vi "HFRR ADV v040 new software.vi"() -> ()   [LabVIEW 2025] (continued)
          frame False {
          }
          frame True {
            n1303 = Not(x=w1625) -> (.not. x?=w1624:bool)
            n1304 = local write "LIVE FEED MIN TEMP"(w1624) -> ()
            n1305 = call "CAMERA LIVE FEED FGV.vi"("Enum - Menu"=CAMERA_LIVE_FEED_ENUM."CAMERA MINIMIZE") -> ()  [unwired: 9 in, 2 out]
          }
        }
        n1306 = local write "CAMERA ROI MAX TEMP"(TRUE ("CAMERA ROI MAX TEMP")) -> ()
        n1307 = case shown="True" w1616 {
          selector: w1616 -> [_ w1622]
          frame False {
          }
          frame True {
            n1308 = Not(x=w1622) -> (.not. x?=w1621:bool)
            n1309 = local write "CAMERA ROI MIN TEMP"(w1621) -> ()
            n1310 = call "IMAGE ANALYSIS.vi"("Enum"=POST_ANALYSIS_ENUM."MINIMIZE UI") -> ()  [unwired: 9 in, 2 out]
          }
        }
      }
    }
    n1311 = local read "Auto Start Test"() -> (w1363:bool)
    n1312 = case shown="True" "sign in temp" {
      frame False {
      }
      frame True {
        w1398 = 1 ("y")
        n1313 = local read "USERNAME"() -> (w1404:string)
        n1314 = local read "USER ID"() -> (w1401:string)
        n1315 = call <vilib>:"Trim Whitespace.vi"("string"=w1404) -> ("trimmed string"=w1403:string)  [unwired: 1 in]
        n1316 = call <vilib>:"Trim Whitespace.vi"("string"=w1401) -> ("trimmed string"=w1402:string)  [unwired: 1 in]
        n1317 = String Length(string=w1403) -> (length=w1400:i32)
        n1318 = String Length(string=w1402) -> (length=w1399:i32)
        n1319 = Greater?(x=w1400, y=w1398) -> (0:w1397:bool)
        n1320 = Greater?(x=w1399, y=w1398) -> (0:w1396:bool)
        n1321 = And(x=w1397, y=w1396) -> (x .and. y?=w1395:bool)
        n1322 = case shown="True" w1395 {
          frame False {
            n1323 = property on="Sign In" class="Bool (strict)"("DisabledEnum"=T19."Disabled" ("Disabled")) -> ()  [unwired: 2 in, 2 out]
          }
          frame True {
            n1324 = property on="Sign In" class="Bool (strict)"("DisabledEnum"=T19."Enabled" ("Disabled")) -> ()  [unwired: 2 in, 2 out]
          }
        }
      }
    }
    n1325 = local read "Air Temperature"() -> (w1380:bool)
    n1326 = local read "Coefficient Of Friction"() -> (w1381:bool)
    n1327 = case shown="False" w1363 {
      frame False {
        n1328 = local read "Auto stop temp"() -> (w1392:bool)
        n1329 = case shown="True" w1392 {
          frame False {
          }
          frame True {
            n1330 = local write "Auto Start Temp"(FALSE ("Auto Start Temp")) -> ()
          }
        }
      }
      frame True {
        "Auto stop temp" <- TRUE ("Auto stop temp")
      }
    }
    n1331 = local read "Humidity 2"() -> (w1379:bool)
    n1332 = case shown="\"HOME\"" w1389 {
      frame "HOME" {
        n1333 = local write "main tab sub"(enum32{"Page 1", "Page 2"}."Page 1" ("main tab sub")) -> ()
      }
      frame Default {
        n1334 = local write "main tab sub"(enum32{"Page 1", "Page 2"}."Page 2" ("main tab sub")) -> ()
      }
    }
    n1335 = case shown="True" w1388 {
      selector: w1388 -> [_ w1741]
      frame False {
      }
      frame True {
        n1336 = Not(x=w1741) -> (.not. x?=w1740:bool)
        n1337 = local write "Sign In"(w1740) -> ()
        n1338 = local write "Main Dashboard Buttons"(T26."Test Setup" ("Main Dashboard Buttons")) -> ()
      }
    }
    n1339 = case shown="\"Numeric Display\", Default" "Num/Graph" {
      frame "Numeric Display", Default {
        n1340 = property on="Single/Multiple" class="RadioBtnsControl (strict)"("Visible"=FALSE) -> ()  [unwired: 2 in, 2 out]
        n1341 = property on="Single - Graph" class="Ring (strict)"("Visible"=FALSE) -> ()  [unwired: 2 in, 2 out]
        n1342 = local write "Main Tab Display"(T4."Dashboard 1" ("Main Tab Display")) -> ()
      }
      frame "Graph Display" {
        n1343 = property on="Single/Multiple" class="RadioBtnsControl (strict)"("Visible"=TRUE) -> ()  [unwired: 2 in, 2 out]
        n1344 = case shown="\"Multiple\"" "Single/Multiple" {
          frame "Single ", Default {
            n1345 = property on="Single - Graph" class="Ring (strict)"("Visible"=TRUE) -> ()  [unwired: 2 in, 2 out]
            n1346 = local write "Main Tab Display"(T4."Dashboard 3" ("Main Tab Display")) -> ()
          }
          frame "Multiple" {
            n1347 = property on="Single - Graph" class="Ring (strict)"("Visible"=FALSE) -> ()  [unwired: 2 in, 2 out]
            n1348 = local write "Main Tab Display"(T4."Dashboard 2" ("Main Tab Display")) -> ()
          }
        }
      }
    }
    n1349 = local read "Stroke"() -> (w1378:bool)
    n1350 = local read "USERNAME"() -> (w1383:string)
    n1351 = case shown="True" w1381 {
      selector: w1381 -> [_ w1665]
      frame False {
      }
      frame True {
        n1352 = Not(x=w1665) -> (.not. x?=w1664:bool)
        n1353 = local write "Coefficient Of Friction"(w1664) -> ()
        n1354 = local write "Tab Control 2"(T6."Coefficient Of Friction" ("Tab Control 2")) -> ()
      }
    }
    n1355 = case shown="True" w1380 {
      selector: w1380 -> [_ w1662]
      frame False {
      }
      frame True {
        n1356 = Not(x=w1662) -> (.not. x?=w1660:bool)
        n1357 = local write "Air Temperature"(w1660) -> ()
        n1358 = local write "Tab Control 2"(T6."Air Temperature" ("Tab Control 2")) -> ()
      }
    }
    n1359 = case shown="True" w1378 {
      selector: w1378 -> [_ w1656]
      frame False {
      }
      frame True {
        n1360 = Not(x=w1656) -> (.not. x?=w1654:bool)
        n1361 = local write "Stroke"(w1654) -> ()
        n1362 = local write "Tab Control 2"(T6."Stroke" ("Tab Control 2")) -> ()
      }
    }
    n1363 = local write "tested by"(w1383) -> ()
    n1364 = case shown="True" w1379 {
      selector: w1379 -> [_ w1659]
      frame False {
      }
      frame True {
        n1365 = Not(x=w1659) -> (.not. x?=w1657:bool)
        n1366 = local write "Humidity 2"(w1657) -> ()
        n1367 = local write "Tab Control 2"(T6."Humidity" ("Tab Control 2")) -> ()
      }
    }
    n1368 = case shown="\"Calibration\"" "Main Dashboard Buttons" {
      tunnel: [T2."HOME" ("Main Tab") T2."Test Setup" ("Main Tab") T2."Acquire" ("Main Tab") T2."Adv Scar" ("Main Tab") T2."Adv Scar Report" ("Main Tab") T2."Compare Files" ("Main Tab") T2."Calibration" ("Main Tab") T2."About" ("Main Tab") T2."Advance" ("Main Tab")] -> w1362
      frame "Home", Default {
      }
      frame "Test Setup" {
      }
      frame "Dashboard" {
      }
      frame "Imaging" {
      }
      frame "Report" {
      }
      frame "Analysis" {
      }
      frame "Calibration" {
      }
      frame "About" {
      }
      frame "Advance" {
      }
    }
    n1369 = Wait (ms)(milliseconds to wait=u32 100) -> ()  [unwired: 1 out]
    n1370 = local read "Main Tab Display"() -> (w1382:T4)
    n1371 = local write "Main Tab"(w1362) -> ()
    n1372 = case shown="\"Dashboard 3\"" w1382 {
      frame "Dashboard 1", Default {
        n1373 = property on="Reset Graph" class="Bool (strict)"("Visible"=FALSE) -> ()  [unwired: 2 in, 2 out]
      }
      frame "Dashboard 2" {
        n1374 = property on="Reset Graph" class="Bool (strict)"("Visible"=TRUE) -> ()  [unwired: 2 in, 2 out]
      }
      frame "Dashboard 3" {
        n1375 = property on="Reset Graph" class="Bool (strict)"("Visible"=TRUE) -> ()  [unwired: 2 in, 2 out]
      }
    }
    n1376 = local read "SCAR MEASURMENT"() -> (w1370:enum32{"Auto Scar", "Manual Scar"})
    n1377 = local read "Humidity"() -> (w1384:bool)
    n1378 = local read "Cap Live Image"() -> (w1367:bool)
    n1379 = local read "Sample Temperature"() -> (w1377:bool)
    n1380 = local read "Air Temp vs Humidity"() -> (w1375:bool)
    n1381 = local read "Frequency"() -> (w1376:bool)
    n1382 = case shown="False" w1384 {
      frame False {
        n1383 = local write "Humidity On Command"(TRUE ("Humidity On Command")) -> ()
        n1384 = case shown="True" "Humidity Off Command" {
          selector: "Humidity Off Command" -> [_ w1672]
          frame False {
          }
          frame True {
            n1385 = stacked-sequence {
              frame #0 {
                n1386 = local write "HUMIDITY CLEAR"(TRUE ("HUMIDITY CLEAR")) -> ()
              }
              frame #1 {
                n1387 = Wait (ms)(milliseconds to wait=u32 500) -> ()  [unwired: 1 out]
              }
              frame #2 {
                n1388 = local read "WriteHumidity"() -> (w1676:string[])
                n1389 = Insert Into Array(array=w1676, new element="R;1" ("new element/subarray")) -> (w1675:string[])  [unwired: 1 in]
                n1390 = local write "WriteHumidity"(w1675) -> ()
              }
              frame #3 {
                n1391 = Wait (ms)(milliseconds to wait=u32 500) -> ()  [unwired: 1 out]
              }
              frame #4 {
                n1392 = local read "WriteHumidity"() -> (w1679:string[])
                n1393 = local read "EVENT LOG"() -> (w1683:string)
                n1394 = call "Event Log.vi"("Content"="Humidity Control Off" ("string"), "EVENT LOG"=w1683) -> ("EVENT LOG"=w1684:string)  [unwired: 8 in, 1 out]
                n1395 = local write "EVENT LOG"(w1684) -> ()
                n1396 = Insert Into Array(array=w1679, new element="R;1" ("new element/subarray")) -> (w1680:string[])  [unwired: 1 in]
                n1397 = local write "WriteHumidity"(w1680) -> ()
              }
            }
            n1398 = Not(x=w1672) -> (.not. x?=w1671:bool)
            n1399 = local write "Humidity Off Command"(w1671) -> ()
          }
        }
      }
      frame True {
        n1400 = local write "Humidity Off Command"(TRUE ("Humidity Off Command")) -> ()
        n1401 = case shown="True" "Humidity On Command" {
          selector: "Humidity On Command" -> [_ w1688]
          frame False {
          }
          frame True {
            n1402 = stacked-sequence {
              frame #0 {
                n1403 = local read "Set Rh"() -> (w1694:dbl)
                n1404 = local read "WriteHumidity"() -> (w1690:string[])
                n1405 = Number To Fractional String(number=w1694, precision (6)=i16 2) -> (F-format string=w1695:string)  [unwired: 2 in]
                n1406 = Concatenate Strings("M;" ("new element/subarray"), w1695) -> (w1693:string)
                n1407 = Insert Into Array(array=w1690, new element=w1693) -> (w1689:string[])  [unwired: 1 in]
                n1408 = local write "WriteHumidity"(w1689) -> ()
              }
              frame #1 {
                n1409 = Wait (ms)(milliseconds to wait=u32 500) -> ()  [unwired: 1 out]
              }
              frame #2 {
                n1410 = local read "WriteHumidity"() -> (w1698:string[])
                n1411 = local read "Set Rh"() -> (w1702:dbl)
                n1412 = Number To Fractional String(number=w1702, precision (6)=i16 2) -> (F-format string=w1703:string)  [unwired: 2 in]
                n1413 = Concatenate Strings("M;" ("new element/subarray"), w1703) -> (w1701:string)
                n1414 = Insert Into Array(array=w1698, new element=w1701) -> (w1697:string[])  [unwired: 1 in]
                n1415 = local write "WriteHumidity"(w1697) -> ()
              }
              frame #3 {
                n1416 = Wait (ms)(milliseconds to wait=u32 500) -> ()  [unwired: 1 out]
              }
              frame #4 {
                (unwired) "% RH" ("string")
                (unwired) i16 2 ("precision (6)")
                (unwired) "M;" ("new element/subarray")
                n1417 = local read "Set Rh"() -> (w1712:dbl)
                n1418 = local read "WriteHumidity"() -> (w1705:string[])
                n1419 = Number To Fractional String(number=w1712, precision (6)=i16 2) -> (F-format string=w1709:string)  [unwired: 2 in]
                n1420 = Concatenate Strings("M;" ("new element/subarray"), w1709) -> (w1713:string)
                n1421 = Concatenate Strings("Humidity Set to : " ("string"), w1709, "% RH" ("string")) -> (w1707:string)
                n1422 = Insert Into Array(array=w1705, new element=w1713) -> (w1706:string[])  [unwired: 1 in]
                n1423 = disable-structure shown="Enabled" {
                  frame Enabled {
                    n1424 = local read "EVENT LOG"() -> (w1716:string)
                    n1425 = call "Event Log.vi"("Content"="Humidity Control On", "EVENT LOG"=w1716) -> ("EVENT LOG"=w1717:string)  [unwired: 8 in, 1 out]
                    n1426 = local write "EVENT LOG"(w1717) -> ()
                  }
                  frame Disabled {
                  }
                }
                n1427 = disable-structure shown="Enabled" {
                  disable-tunnel: w1707 -> [_ _]
                  frame Enabled {
                    n1428 = local read "EVENT LOG"() -> (w1719:string)
                    n1429 = call "Event Log.vi"("Content"="Humidity Control On", "EVENT LOG"=w1719) -> ("EVENT LOG"=w1720:string)  [unwired: 8 in, 1 out]
                    n1430 = local write "EVENT LOG"(w1720) -> ()
                  }
                  frame Disabled {
                  }
                }
                n1431 = local write "WriteHumidity"(w1706) -> ()
              }
            }
            n1432 = Not(x=w1688) -> (.not. x?=w1687:bool)
            n1433 = local write "Humidity On Command"(w1687) -> ()
          }
        }
      }
    }
    n1434 = Equal?(x=w1370, y=enum32{"Auto Scar", "Manual Scar"}."Auto Scar" ("SCAR MEASURMENT")) -> (x = y?=w1366:bool)
    n1435 = local read "TEST STANDARD"() -> (w1373:T3)
    n1436 = And(x=w1367, y=w1366) -> (x .and. y?=w1368:bool)
    n1437 = case shown="True" w1368 {
      selector: w1368 -> [_ w1471]
      tunnel: errorcluster {"status"=FALSE, "code"=0, "source"=""} ("error in (no error) 3") -> [_ w1472]
      frame False {
      }
      frame True {
        n1438 = stacked-sequence {
          tunnel: w1472 -> [_ _ _ _ _ _ _ w1520]
          tunnel: w1471 -> [_ _ _ _ _ w1501 _ _]
          frame #0 {
            n1439 = call "CAMERA LIVE FEED FGV.vi"("Enum - Menu"=CAMERA_LIVE_FEED_ENUM."CAMERA MINIMIZE") -> ()  [unwired: 9 in, 2 out]
          }
          frame #1 {
            n1440 = property on="Auto Scar Check  2" class="Clust (strict)"("Visible"=TRUE) -> ()  [unwired: 2 in, 2 out]
          }
          frame #2 {
            n1441 = String To Path(string="C:\\LAB-IQ\\Image Calibrate v01.dcf") -> (path=w1477:path)
            n1442 = Open/Create/Replace File ("Open File")(file path (use dialog)=w1477) -> (refnum out=w1478:refnum<file>)  [unwired: 5 in, 2 out]
            n1443 = for {
              N: 4 -> [_]
              tunnel: w1478 -> [w1484]
              i -> [w1480]
              n1444 = Read from Text File ("Read File")(file (use dialog)=w1484) -> (text=w1485:string)  [unwired: 3 in, 3 out]
              n1445 = String Subset(string=w1485, offset (0)=6, length (rest)=10 ("length (rest)")) -> (substring=w1481:string)
              n1446 = Fract/Exp String To Number(string=w1481) -> (number=w1479:dbl)  [unwired: 3 in, 1 out]
              n1447 = case shown="0" w1480 {
                tunnel: w1479 -> [w1486 w1487 _ w1488 _]
                frame 0 {
                  "5x Gain" <- w1486
                }
                frame 1 {
                  "10x Gain" <- w1487
                }
                frame 2 {
                }
                frame 3 {
                  "100x gain" <- w1488
                }
                frame 4, Default {
                }
              }
            }
          }
          frame #3 {
            n1448 = local read "FILE 3"() -> (w1494:string)
            n1449 = call <vilib>:"Trim Whitespace.vi"("string"="C:\\LAB-IQ\\images\\") -> ("trimmed string"=w1496:string)  [unwired: 1 in]
            n1450 = String To Path(string=w1496) -> (path=w1495:path)
            n1451 = Concatenate Strings(w1494, ".png" ("string")) -> (w1493:string)
            n1452 = Build Path(base path=w1495, name or relative path=w1493) -> (appended path=w1491:path)
            "Image path" <- w1491
            n1453 = Path To String(path=w1491) -> (string=w1490:string)
            n1454 = call "CAMERA LIVE FEED FGV.vi"("Enum - Menu"=CAMERA_LIVE_FEED_ENUM."CAMERA SAVE", "Image Path"=w1490) -> ()  [unwired: 8 in, 2 out]
          }
          frame #4 {
            n1455 = One Button Dialog(message="Image saved successfully") -> ()  [unwired: 1 in, 1 out]
          }
          frame #5 {
            n1456 = local read "TEST STANDARD"() -> (w1500:T3)
            n1457 = local read "Magnification len live scar"() -> (w1512:string)
            n1458 = Not(x=w1501) -> (.not. x?=w1502:bool)
            n1459 = local write "Cap Live Image"(w1502) -> ()
            n1460 = case shown="\"ISO 12156\"" w1500 {
              tunnel: ["ASTM D6079" "ISO 12156"] -> w1499
              frame "ASTM D6079", Default {
              }
              frame "ISO 12156" {
              }
            }
            n1461 = case shown="\"5x\", Default" w1512 {
              tunnel: [w1515 w1516] -> w1511
              frame "5x", Default {
                n1462 = local read "5x Gain"() -> (w1515:dbl)
              }
              frame "10x" {
                # "5x"
                n1463 = local read "10x Gain"() -> (w1516:dbl)
              }
            }
            n1464 = local read "Image path"() -> (w1510:path)
            n1465 = local read "FILE 3"() -> (w1503:string)
            n1466 = call "EDGE DETCTION.vi"("GAIN VALUE"=w1511, "Image Path"=w1510) -> ("error out"=w1509:errorcluster, "return value"=w1508:cluster{string, string, dbl, dbl, dbl})  [unwired: 8 in]
            n1467 = Bundle By Name(cluster=T27 {"File Name"="", "Test Method"="", "Operator"="", "Fuel Description"="", "Date and time"=""} ("Main Ref"), "File Name"=w1503, "Test Method"=w1499) -> (w1504:T27)
            n1468 = call "duf file read.vi"("error in (no error)"=w1509, "Main Ref"=w1504) -> ("error out"=w1507:errorcluster, "Main Ref 2"=w1505:T27)  [unwired: 8 in]
            n1469 = call "EDGE DETECTION REPORT.vi"("error in (no error)"=w1507, "return value 2"=w1508, "Main Ref"=w1505) -> ()  [unwired: 8 in, 1 out]
          }
          frame #6 {
            n1470 = property on="Auto Scar Check  2" class="Clust (strict)"("Visible"=FALSE) -> ()  [unwired: 2 in, 2 out]
          }
          frame #7 {
            n1471 = call "CAMERA LIVE FEED FGV.vi"("Enum - Menu"=CAMERA_LIVE_FEED_ENUM."CAMERA MINIMIZE", "error in (no error)"=w1520) -> ()  [unwired: 8 in, 2 out]
            n1472 = local write "Main Dashboard Buttons"(T1."Home" ("Main Dashboard Buttons")) -> ()
            n1473 = local write "Main Tab"(T2."HOME" ("Main Tab")) -> ()
          }
        }
      }
    }
    n1474 = local read "Heater Button"() -> (w1374:bool)
    n1475 = case shown="True" w1376 {
      selector: w1376 -> [_ w1650]
      frame False {
      }
      frame True {
        n1476 = Not(x=w1650) -> (.not. x?=w1648:bool)
        n1477 = local write "Frequency"(w1648) -> ()
        n1478 = local write "Tab Control 2"(T6."Frequency" ("Tab Control 2")) -> ()
      }
    }
    n1479 = case shown="True" w1375 {
      selector: w1375 -> [_ w1647]
      frame False {
      }
      frame True {
        n1480 = Not(x=w1647) -> (.not. x?=w1645:bool)
        n1481 = local write "Air Temp vs Humidity"(w1645) -> ()
        n1482 = local write "Tab Control 2"(T6."Air Temp vs Rh" ("Tab Control 2")) -> ()
      }
    }
    n1483 = case shown="True" w1377 {
      selector: w1377 -> [_ w1653]
      frame False {
      }
      frame True {
        n1484 = Not(x=w1653) -> (.not. x?=w1651:bool)
        n1485 = local write "Sample Temperature"(w1651) -> ()
        n1486 = local write "Tab Control 2"(T6."Sample Temperature" ("Tab Control 2")) -> ()
      }
    }
    n1487 = case shown="\"Custom\"" w1373 {
      frame "ASTM D6079", Default {
        w1626 = "ASTM D6079 TEST CONDITIONS" ("Standard 2")
        n1488 = local write "Standard 2"(w1626) -> ()
        n1489 = local write "Standard"(w1626) -> ()
      }
      frame "ISO 12156" {
        w1627 = "ISO 12156 TEST CONDITIONS" ("Standard 2")
        n1490 = local write "Standard 2"(w1627) -> ()
        n1491 = local write "Standard"(w1627) -> ()
      }
      frame "CEC F-096-A-06" {
        w1628 = "CEC F-096-A-06 TEST CONDITIONS" ("Standard 2")
        n1492 = local write "Standard 2"(w1628) -> ()
        n1493 = local write "Standard"(w1628) -> ()
      }
      frame "Custom" {
        w1629 = "CUSTOM TEST CONDITIONS" ("Standard 2")
        n1494 = local write "Standard 2"(w1629) -> ()
        n1495 = local write "Standard"(w1629) -> ()
      }
    }
    n1496 = case shown="True" w1374 {
      frame False {
        n1497 = local write "Temperature On Command"(TRUE ("Temperature On Command")) -> ()
        n1498 = case shown="True" "Temperature Off Command" {
          selector: "Temperature Off Command" -> [_ w1633]
          frame False {
          }
          frame True {
            n1499 = Not(x=w1633) -> (.not. x?=w1632:bool)
            n1500 = local read "EVENT LOG"() -> (w1636:string)
            n1501 = local write "Temperature Off Command"(w1632) -> ()
            n1502 = call "Event Log.vi"("Content"="Heater Off", "EVENT LOG"=w1636) -> ("EVENT LOG"=w1635:string)  [unwired: 8 in, 1 out]
            n1503 = local write "EVENT LOG"(w1635) -> ()
          }
        }
      }
      frame True {
        n1504 = local write "Temperature Off Command"(TRUE ("Temperature Off Command")) -> ()
        n1505 = case shown="True" "Temperature On Command" {
          selector: "Temperature On Command" -> [_ w1640]
          frame False {
          }
          frame True {
            n1506 = Not(x=w1640) -> (.not. x?=w1639:bool)
            n1507 = local write "Temperature On Command"(w1639) -> ()
            n1508 = disable-structure shown="Enabled" {
              disable-tunnel: "Heater On" -> [w1642 _]
              frame Enabled {
                n1509 = local read "EVENT LOG"() -> (w1643:string)
                n1510 = call "Event Log.vi"("Content"=w1642, "EVENT LOG"=w1643) -> ("EVENT LOG"=w1644:string)  [unwired: 8 in, 1 out]
                n1511 = local write "EVENT LOG"(w1644) -> ()
              }
              frame Disabled {
              }
            }
          }
        }
      }
    }
    n1512 = local read "Main Tab"() -> (w1365:T2)
    n1513 = case shown="\"About\"" w1365 {
      frame "HOME", Default {
        w1407 = T19."Enabled" ("Disabled")
        n1514 = local read "Service Password enable"() -> (w1409:bool)
        n1515 = property on="Imaging" class="Bool (strict)"("DisabledEnum"=w1407) -> ()  [unwired: 2 in, 2 out]
        n1516 = property on="Dashboard" class="Bool (strict)"("DisabledEnum"=w1407) -> ()  [unwired: 2 in, 2 out]
        n1517 = property on="Test Setup" class="Bool (strict)"("DisabledEnum"=w1407) -> ()  [unwired: 2 in, 2 out]
        n1518 = property on="Analysis" class="Bool (strict)"("DisabledEnum"=w1407) -> ()  [unwired: 2 in, 2 out]
        n1519 = property on="Home" class="Bool (strict)"("DisabledEnum"=w1407) -> ()  [unwired: 2 in, 2 out]
        n1520 = property on="Report" class="Bool (strict)"("DisabledEnum"=w1407) -> ()  [unwired: 2 in, 2 out]
        n1521 = property on="Main Dashboard Buttons" class="RadioBtnsControl (strict)"("DisabledEnum"=w1407) -> ()  [unwired: 2 in, 2 out]
        n1522 = property on="Calibration" class="Bool (strict)"("DisabledEnum"=w1407) -> ()  [unwired: 2 in, 2 out]
        n1523 = case shown="True" w1409 {
          tunnel: [T19."Disabled" ("Disabled") T19."Enabled" ("Disabled")] -> w1408
          frame False {
          }
          frame True {
          }
        }
        n1524 = property on="About" class="Bool (strict)"("DisabledEnum"=w1408) -> ()  [unwired: 2 in, 2 out]
      }
      frame "Test Setup" {
        w1414 = T19."Enabled" ("Disabled")
        n1525 = local read "Service Password enable"() -> (w1413:bool)
        n1526 = property on="Dashboard" class="Bool (strict)"("DisabledEnum"=T19."Disabled" ("Disabled")) -> ()  [unwired: 2 in, 2 out]
        n1527 = property on="Imaging" class="Bool (strict)"("DisabledEnum"=w1414) -> ()  [unwired: 2 in, 2 out]
        n1528 = property on="Analysis" class="Bool (strict)"("DisabledEnum"=w1414) -> ()  [unwired: 2 in, 2 out]
        n1529 = property on="Home" class="Bool (strict)"("DisabledEnum"=w1414) -> ()  [unwired: 2 in, 2 out]
        n1530 = property on="Report" class="Bool (strict)"("DisabledEnum"=w1414) -> ()  [unwired: 2 in, 2 out]
        n1531 = property on="Test Setup" class="Bool (strict)"("DisabledEnum"=w1414) -> ()  [unwired: 2 in, 2 out]
        n1532 = case shown="True" w1413 {
          tunnel: [T19."Disabled" ("Disabled") T19."Enabled" ("Disabled")] -> w1412
          frame False {
          }
          frame True {
          }
        }
        n1533 = property on="About" class="Bool (strict)"("DisabledEnum"=w1412) -> ()  [unwired: 2 in, 2 out]
      }
      frame "Adv Scar" {
        w1421 = T19."Enabled" ("Disabled")
        n1534 = property on="Dashboard" class="Bool (strict)"("DisabledEnum"=T19."Disabled" ("Disabled")) -> ()  [unwired: 2 in, 2 out]
        n1535 = property on="Imaging" class="Bool (strict)"("DisabledEnum"=w1421) -> ()  [unwired: 2 in, 2 out]
        n1536 = property on="Analysis" class="Bool (strict)"("DisabledEnum"=w1421) -> ()  [unwired: 2 in, 2 out]
        n1537 = property on="Home" class="Bool (strict)"("DisabledEnum"=w1421) -> ()  [unwired: 2 in, 2 out]
        n1538 = property on="Report" class="Bool (strict)"("DisabledEnum"=w1421) -> ()  [unwired: 2 in, 2 out]
        n1539 = property on="Test Setup" class="Bool (strict)"("DisabledEnum"=w1421) -> ()  [unwired: 2 in, 2 out]
        n1540 = local read "Service Password enable"() -> (w1419:bool)
        n1541 = case shown="True" w1419 {
          tunnel: [T19."Disabled" ("Disabled") T19."Enabled" ("Disabled")] -> w1418
          frame False {
          }
          frame True {
          }
        }
        n1542 = property on="About" class="Bool (strict)"("DisabledEnum"=w1418) -> ()  [unwired: 2 in, 2 out]
      }
      frame "Calibration" {
        w1424 = T19."Enabled" ("Disabled")
        n1543 = property on="Dashboard" class="Bool (strict)"("DisabledEnum"=T19."Disabled" ("Disabled")) -> ()  [unwired: 2 in, 2 out]
        n1544 = property on="Imaging" class="Bool (strict)"("DisabledEnum"=w1424) -> ()  [unwired: 2 in, 2 out]
        n1545 = property on="Analysis" class="Bool (strict)"("DisabledEnum"=w1424) -> ()  [unwired: 2 in, 2 out]
        n1546 = property on="Home" class="Bool (strict)"("DisabledEnum"=w1424) -> ()  [unwired: 2 in, 2 out]
        n1547 = property on="Report" class="Bool (strict)"("DisabledEnum"=w1424) -> ()  [unwired: 2 in, 2 out]
        n1548 = property on="Test Setup" class="Bool (strict)"("DisabledEnum"=w1424) -> ()  [unwired: 2 in, 2 out]
        n1549 = local read "Service Password enable"() -> (w1426:bool)
        n1550 = property on="Calibration" class="Bool (strict)"("DisabledEnum"=w1424) -> ()  [unwired: 2 in, 2 out]
        n1551 = case shown="True" w1426 {
          tunnel: [T19."Disabled" ("Disabled") T19."Enabled" ("Disabled")] -> w1425
          frame False {
          }
          frame True {
          }
        }
        n1552 = property on="About" class="Bool (strict)"("DisabledEnum"=w1425) -> ()  [unwired: 2 in, 2 out]
      }
      frame "Adv Scar Report" {
        w1432 = T19."Enabled" ("Disabled")
        n1553 = property on="Dashboard" class="Bool (strict)"("DisabledEnum"=T19."Disabled" ("Disabled")) -> ()  [unwired: 2 in, 2 out]
        n1554 = property on="Imaging" class="Bool (strict)"("DisabledEnum"=w1432) -> ()  [unwired: 2 in, 2 out]
        n1555 = property on="Analysis" class="Bool (strict)"("DisabledEnum"=w1432) -> ()  [unwired: 2 in, 2 out]
        n1556 = property on="Home" class="Bool (strict)"("DisabledEnum"=w1432) -> ()  [unwired: 2 in, 2 out]
        n1557 = property on="Report" class="Bool (strict)"("DisabledEnum"=w1432) -> ()  [unwired: 2 in, 2 out]
        n1558 = property on="Test Setup" class="Bool (strict)"("DisabledEnum"=w1432) -> ()  [unwired: 2 in, 2 out]
        n1559 = local read "Service Password enable"() -> (w1431:bool)
        n1560 = case shown="True" w1431 {
          tunnel: [T19."Disabled" ("Disabled") T19."Enabled" ("Disabled")] -> w1430
          frame False {
          }
          frame True {
          }
        }
        n1561 = property on="About" class="Bool (strict)"("DisabledEnum"=w1430) -> ()  [unwired: 2 in, 2 out]
      }
      frame "Compare Files" {
        w1438 = T19."Enabled" ("Disabled")
        n1562 = local read "Service Password enable"() -> (w1437:bool)
        n1563 = property on="Dashboard" class="Bool (strict)"("DisabledEnum"=T19."Disabled" ("Disabled")) -> ()  [unwired: 2 in, 2 out]
        n1564 = property on="Imaging" class="Bool (strict)"("DisabledEnum"=w1438) -> ()  [unwired: 2 in, 2 out]
        n1565 = property on="Analysis" class="Bool (strict)"("DisabledEnum"=w1438) -> ()  [unwired: 2 in, 2 out]
        n1566 = property on="Home" class="Bool (strict)"("DisabledEnum"=w1438) -> ()  [unwired: 2 in, 2 out]
        n1567 = property on="Report" class="Bool (strict)"("DisabledEnum"=w1438) -> ()  [unwired: 2 in, 2 out]
        n1568 = property on="Test Setup" class="Bool (strict)"("DisabledEnum"=w1438) -> ()  [unwired: 2 in, 2 out]
        n1569 = case shown="True" w1437 {
          tunnel: [T19."Disabled" ("Disabled") T19."Enabled" ("Disabled")] -> w1436
          frame False {
          }
          frame True {
          }
        }
        n1570 = property on="About" class="Bool (strict)"("DisabledEnum"=w1436) -> ()  [unwired: 2 in, 2 out]
      }
      frame "Acquire" {
        n1571 = local read "Service Password enable"() -> (w1443:bool)
        n1572 = property on="Test Setup" class="Bool (strict)"("DisabledEnum"=T19."Disabled" ("Disabled")) -> ()  [unwired: 2 in, 2 out]
        n1573 = local read "Auto Start Test"() -> (w1445:bool)
        n1574 = local read "RUN"() -> (w1447:bool)
        n1575 = case shown="True" w1443 {
          tunnel: [T19."Disabled" ("Disabled") T19."Enabled" ("Disabled")] -> w1444
          frame False {
          }
          frame True {
          }
        }
        n1576 = Or(x=w1447, y=w1445) -> (x .or. y?=w1446:bool)
        n1577 = case shown="True" w1446 {
          tunnel: [T19."Enabled" ("Disabled") T19."Disabled" ("Disabled")] -> w1442
          frame False {
          }
          frame True {
          }
        }
        n1578 = property on="About" class="Bool (strict)"("DisabledEnum"=w1444) -> ()  [unwired: 2 in, 2 out]
        n1579 = property on="Imaging" class="Bool (strict)"("DisabledEnum"=w1442) -> ()  [unwired: 2 in, 2 out]
        n1580 = property on="Dashboard" class="Bool (strict)"("DisabledEnum"=w1442) -> ()  [unwired: 2 in, 2 out]
        n1581 = property on="Analysis" class="Bool (strict)"("DisabledEnum"=w1442) -> ()  [unwired: 2 in, 2 out]
        n1582 = property on="Home" class="Bool (strict)"("DisabledEnum"=w1442) -> ()  [unwired: 2 in, 2 out]
        n1583 = property on="Report" class="Bool (strict)"("DisabledEnum"=w1442) -> ()  [unwired: 2 in, 2 out]
        n1584 = property on="Calibration" class="Bool (strict)"("DisabledEnum"=w1442) -> ()  [unwired: 2 in, 2 out]
      }
      frame "About" {
        n1585 = local read "FILE"() -> (w1461:string)
        n1586 = local read "TEST FILE NAM,E SAVED"() -> (w1454:bool)
        n1587 = call <vilib>:"Trim Whitespace.vi"("string"=w1461) -> ("trimmed string"=w1460:string)  [unwired: 1 in]
        n1588 = local read "Auto Start Test"() -> (w1464:bool)
        n1589 = String Length(string=w1460) -> (length=w1459:i32)
        n1590 = Greater?(x=w1459, y=1) -> (0:w1456:bool)
        n1591 = And(x=w1456, y=w1454) -> (x .and. y?=w1455:bool)
        n1592 = local read "RUN"() -> (w1466:bool)
        n1593 = case shown="True" w1455 {
          tunnel: [T19."Disabled" ("Disabled") T19."Enabled" ("Disabled")] -> w1457
          frame False {
          }
          frame True {
          }
        }
        n1594 = Or(x=w1466, y=w1464) -> (x .or. y?=w1465:bool)
        n1595 = property on="About" class="Bool (strict)"("DisabledEnum"=T19."Enabled" ("Disabled")) -> ()  [unwired: 2 in, 2 out]
        n1596 = case shown="False" w1465 {
          tunnel: [T19."Enabled" ("Disabled") T19."Disabled" ("Disabled")] -> w1463
          frame False {
          }
          frame True {
          }
        }
        n1597 = property on="Dashboard" class="Bool (strict)"("DisabledEnum"=w1457) -> ()  [unwired: 2 in, 2 out]
        n1598 = property on="Test Setup" class="Bool (strict)"("DisabledEnum"=T19."Disabled" ("Disabled")) -> ()  [unwired: 2 in, 2 out]
        n1599 = property on="Imaging" class="Bool (strict)"("DisabledEnum"=w1463) -> ()  [unwired: 2 in, 2 out]
        n1600 = property on="Analysis" class="Bool (strict)"("DisabledEnum"=w1463) -> ()  [unwired: 2 in, 2 out]
        n1601 = property on="Home" class="Bool (strict)"("DisabledEnum"=w1463) -> ()  [unwired: 2 in, 2 out]
        n1602 = property on="Report" class="Bool (strict)"("DisabledEnum"=w1463) -> ()  [unwired: 2 in, 2 out]
      }
    }
    n1603 = local read "Quit"() -> (w1391:bool)
    "Single" <- "Single - Graph"
  }
  n1604 = disable-structure shown="Disabled" {
    disable-tunnel: [w1745 _] -> w42
    disable-tunnel: _ -> [w1744 _]
    frame Disabled {
      n1605 = while {
        tunnel: w1744 -> [_]
        tunnel: [w1746] -> w1745
        tunnel: [w1747] -> _
        i -> [w1747]
        stop <- w1746 stop-if-true
        w1763 = u16 10 items=["1.0"=10, "1.5"=15, "2.0"=20] ("stop bits (10: 1 bit)")
        n1606 = Wait (ms)(milliseconds to wait=u32 10) -> ()  [unwired: 1 out]
        n1607 = call-poly "VISA Configure Serial Port"("VISA resource name"=refnum<visa-resource-name> "ASRL1::INSTR" ("COM PORT"), "timeout (10sec)"=u32 10, "baud rate (9600)"=u32 57600, "data bits (8)"=u16 8, "stop bits (10: 1 bit)"=w1763) -> ("VISA resource name out"=w1749:refnum<visa-resource-name>, "error out"=w1758:errorcluster)  [unwired: 9 in]
        n1608 = VISA Read(VISA resource name=w1749, byte count=u32 2 ("byte count (0)")) -> (read buffer=w1757:string)  [unwired: 1 in, 3 out]
        n1609 = String Subset(string=w1757, offset (0)=0, length (rest)=2 ("length (rest)")) -> (substring=w1756:string)
        n1610 = Match Pattern(string=w1756, regular expression="<>") -> (offset past match=w1753:i32)  [unwired: 1 in, 3 out]
        n1611 = Greater Or Equal?(x=w1753, y=0) -> (x >= y?=w1748:bool)
        n1612 = case shown="True" w1748 {
          tunnel: w1749 -> [_ w1767]
          tunnel: w1758 -> [_ w1766]
          frame False {
          }
          frame True {
            n1613 = VISA Read(VISA resource name=w1767, byte count=u32 32 ("byte count (0)"), error in (no error)=w1766) -> (read buffer=w1765:string)  [unwired: 3 out]
            n1614 = String Subset(string=w1765, offset (0)=0, length (rest)=8 ("length (rest)")) -> (substring=w1769:string)
            n1615 = String Subset(string=w1765, offset (0)=8, length (rest)=8 ("length (rest)")) -> (substring=w1770:string)
            n1616 = Decimal String To Number(string=w1770) -> (number=w1777:i32)  [unwired: 2 in, 1 out]
            n1617 = Decimal String To Number(string=w1769) -> (number=w1773:i32)  [unwired: 2 in, 1 out]
            n1618 = Divide(x=w1777, y=10000) -> ()  [unwired: 1 out]
            n1619 = Divide(x=w1773, y=1000000) -> ()  [unwired: 1 out]
          }
        }
        n1620 = local read "Quit"() -> (w1746:bool)
      }
    }
    frame Enabled {
    }
  }
  n1621 = Tick Count (ms)() -> (millisecond timer value=w4:u32)
  n1622 = while {
    shift-right: [w1823] -> _
    shift-left: w6 -> [w1827]
    shift-right: [w1822] -> _
    shift-left: w5 -> [w1826]
    shift-right: [w1821] -> _
    shift-left: w6 -> [w1825]
    shift-right: [w1820] -> _
    shift-left: w5 -> [w1824]
    shift-right: [w1818] -> _
    shift-left: w4 -> [w1819]
    shift-right: [w1815] -> _
    shift-left: w3 -> [w1816]
    shift-right: [w1814] -> _
    shift-left: w3 -> [w1817]
    shift-right: [w1807] -> _
    shift-left: w3 -> [w1813]
    shift-right: [w1806] -> _
    shift-left: w3 -> [w1812]
    shift-right: [w1805] -> _
    shift-left: w3 -> [w1811]
    shift-right: [w1804] -> _
    shift-left: w3 -> [w1810]
    shift-right: [w1803] -> _
    shift-left: w3 -> [w1809]
    shift-right: [w1802] -> _
    shift-left: w3 -> [w1808]
    shift-right: [w1801] -> _
    shift-left: w3 -> [w1795]
    shift-right: [w1800] -> _
    shift-left: w3 -> [w1794]
    shift-right: [w1799] -> _
    shift-left: w3 -> [w1793]
    shift-right: [w1798] -> _
    shift-left: w3 -> [w1792]
    shift-right: [w1797] -> _
    shift-left: w3 -> [w1791]
    shift-right: [w1796] -> _
    shift-left: w3 -> [w1790]
    shift-right: [w1781] -> _
    shift-left: w3 -> [w1784]
    shift-right: [w1780] -> _
    shift-left: w3 -> [w1783]
    shift-right: [w1779] -> _
    shift-left: w3 -> [w1782]
    stop <- w1829 stop-if-true
    n1623 = local read "Read UNO"() -> (w1788:string)
    n1624 = local read "Error  2"() -> (w1828:errorcluster)
    n1625 = String Length(string=w1788) -> (length=w1787:i32)
    n1626 = call <vilib>:"Trim Whitespace.vi"("string"=w1788) -> ("trimmed string"=w1789:string)  [unwired: 1 in]
    n1627 = Greater Or Equal?(x=w1787, y=23) -> (x >= y?=w1785:bool)
    n1628 = case shown="No Error" w1828 {
      tunnel: w1827 -> [w1875 w1971]
      tunnel: w1826 -> [w1874 w1970]
      tunnel: w1825 -> [w1873 w1969]
      tunnel: w1824 -> [w1872 w1968]
      tunnel: [w1871 w1971] -> w1823
      tunnel: [w1870 w1970] -> w1822
      tunnel: [w1869 w1969] -> w1821
      tunnel: [w1868 w1968] -> w1820
      tunnel: w1819 -> [w1867 w1967]
      tunnel: [w1866 w1967] -> w1818
      tunnel: w1816 -> [w1865 w1966]
      tunnel: w1817 -> [w1864 w1965]
      tunnel: [w1863 w1966] -> w1815
      tunnel: [w1862 w1965] -> w1814
      tunnel: w1813 -> [w1861 w1964]
      tunnel: w1812 -> [w1860 w1963]
      tunnel: w1811 -> [w1859 w1962]
      tunnel: w1810 -> [w1858 w1961]
      tunnel: w1809 -> [w1857 w1960]
      tunnel: w1808 -> [w1856 w1959]
      tunnel: [w1855 w1964] -> w1807
      tunnel: [w1854 w1963] -> w1806
      tunnel: [w1853 w1962] -> w1805
      tunnel: [w1852 w1961] -> w1804
      tunnel: [w1851 w1960] -> w1803
      tunnel: [w1850 w1959] -> w1802
      tunnel: w1795 -> [w1849 w1958]
      tunnel: [w1848 w1958] -> w1801
      tunnel: [w1847 w1954] -> w1800
      tunnel: [w1846 w1953] -> w1799
      tunnel: [w1845 w1957] -> w1798
      tunnel: [w1844 w1956] -> w1797
      tunnel: [w1843 w1955] -> w1796
      tunnel: w1794 -> [w1842 w1957]
      tunnel: w1793 -> [w1841 w1956]
      tunnel: w1792 -> [w1840 w1955]
      tunnel: w1791 -> [w1839 w1954]
      tunnel: w1790 -> [w1838 w1953]
      tunnel: w1789 -> [w1837 _]
      tunnel: w1785 -> [w1836 _]
      tunnel: w1784 -> [w1835 w1952]
      tunnel: w1783 -> [w1834 w1951]
      tunnel: w1782 -> [w1833 w1950]
      tunnel: [w1832 w1952] -> w1781
      tunnel: [w1831 w1951] -> w1780
      tunnel: [w1830 w1950] -> w1779
      frame No Error {
        n1629 = case shown="True" w1836 {
          tunnel: w1875 -> [w1891 w1943]
          tunnel: w1874 -> [w1890 w1942]
          tunnel: w1873 -> [w1889 w1941]
          tunnel: w1872 -> [w1888 w1940]
          tunnel: [w1891 w1939] -> w1871
          tunnel: [w1890 w1938] -> w1870
          tunnel: [w1889 w1937] -> w1869
          tunnel: [w1888 w1936] -> w1868
          tunnel: w1867 -> [w1887 w1934]
          tunnel: [w1887 w1933] -> w1866
          tunnel: w1865 -> [w1886 w1932]
          tunnel: w1864 -> [w1885 w1931]
          tunnel: [w1886 w1930] -> w1863
          tunnel: [w1885 w1929] -> w1862
          tunnel: w1861 -> [w1884 w1928]
          tunnel: w1860 -> [w1883 w1927]
          tunnel: w1859 -> [w1882 w1926]
          tunnel: w1858 -> [w1881 w1925]
          tunnel: w1857 -> [w1880 w1924]
          tunnel: w1856 -> [w1879 w1923]
          tunnel: [w1884 w1922] -> w1855
          tunnel: [w1883 w1921] -> w1854
          tunnel: [w1882 w1920] -> w1853
          tunnel: [w1881 w1919] -> w1852
          tunnel: [w1880 w1918] -> w1851
          tunnel: [w1879 w1917] -> w1850
          tunnel: w1849 -> [w1897 w1916]
          tunnel: [w1897 w1915] -> w1848
          tunnel: [w1894 w1914] -> w1847
          tunnel: [w1893 w1913] -> w1846
          tunnel: [w1896 w1912] -> w1845
          tunnel: [w1892 w1911] -> w1844
          tunnel: [w1895 w1910] -> w1843
          tunnel: w1842 -> [w1896 w1909]
          tunnel: w1841 -> [w1895 w1908]
          tunnel: w1840 -> [w1894 w1907]
          tunnel: w1839 -> [w1893 w1906]
          tunnel: w1838 -> [w1892 w1905]
          tunnel: w1837 -> [_ w1904]
          tunnel: w1835 -> [w1878 w1903]
          tunnel: w1834 -> [w1877 w1902]
          tunnel: w1833 -> [w1876 w1901]
          tunnel: [w1878 w1900] -> w1832
          tunnel: [w1877 w1899] -> w1831
          tunnel: [w1876 w1898] -> w1830
          frame False {
          }
          frame True {
            n1630 = Tick Count (ms)() -> (millisecond timer value=w1935:u32)
            n1631 = String To Byte Array(string=w1904) -> (unsigned byte array=w1948:u8[])
            n1632 = Array Size(array=w1948) -> (size(s)=w1947:i32)
            n1633 = formula code="// --- INTERNAL VARIABLE DECLARATIONS ---\nint i = 0;\nint k = 0;\nint start_idx = -1;\nint end_idx = -1;\nint phase = 0;\nint sign0 = 1;\nint sign1 = 1;\nint ch0_val = 0;   \nint ch1_val = 0;   \nfloat ch0_raw = 0.0;\nfloat ch1_raw = 0.0;\nfloat temp0 = 0.0;\nfloat temp1 = 0.0;\nfloat ch0_clean = 0.0;\nfloat ch1_clean = 0.0;\n\nint valid_samples = 0; // FIX: Track if we actually parsed new data this window\nfloat max_allowed_bits = 8388607.0; // FIX: Change this to match your ADC max value\n\n// Temporal intermediate variables for calculation smoothing\nfloat raw_p2p_v = 0.0;\nfloat raw_friction = 0.0;\nfloat raw_cof = 0.0;\n\n// Temporal intermediate variables for Piezo voltage translations\nfloat piezo_min_v = 0.0;\nfloat piezo_max_v = 0.0;\n\n// Initialize output variables to current shift register states right away\nout_LVDT_Min_V = in_LVDT_Min_V;\nout_LVDT_Max_V = in_LVDT_Max_V;\nout_LVDT_P2P_V = in_LVDT_P2P_V;\nout_Piezo_P2P = in_Piezo_P2P;\nout_Friction_N = in_Friction_N;\nout_COF = in_COF;\nwindow_ready = 0;\n\n// --- STEP 1: PARSE EVERY STRING IN THE BYTE ARRAY ---\nif (array_size > 2) {\n    for (i = 0; i < array_size - 1; i++) {\n        if (raw_bytes[i] == 42) { // '*' character detected\n            start_idx = i;\n        }\n        \n        // Match standard delimiter sequence \";&\" or end window character\n        if (raw_bytes[i] == 59 && raw_bytes[i+1] == 38 && start_idx != -1) { \n            end_idx = i;\n            ch0_val = 0;\n            ch1_val = 0;\n            sign0 = 1;\n            sign1 = 1;\n            phase = 0; \n\n            for (k = start_idx + 1; k < end_idx; k++) {\n                if (raw_bytes[k] == 45) { // '-' sign\n                    if (phase == 0) sign0 = -1;\n                    else sign1 = -1;\n                }\n                else if (raw_bytes[k] == 43) { // '+' sign\n                    if (phase == 0) sign0 = 1;\n                    else sign1 = 1;\n                }\n                else if (raw_bytes[k] == 59) { // ';' delimiter\n                    phase = 1; \n                }\n                else if (raw_bytes[k] >= 48 && raw_bytes[k] <= 57) { // Numeric ASCII digits\n                    if (phase == 0) {\n                        ch0_val = (ch0_val * 10) + (raw_bytes[k] - 48);\n                    } else {\n                        ch1_val = (ch1_val * 10) + (raw_bytes[k] - 48);\n                    }\n                }\n            }\n\n            // Implicit type conversion\n            ch0_raw = ch0_val * sign0 * 1.0;\n            ch1_raw = ch1_val * sign1 * 1.0;\n\n            // FIX: Sanity check / Hard-clamping to catch sudden massive ASCII noise spikes\n            if (ch0_raw > max_allowed_bits)  ch0_raw = max_allowed_bits;\n            if (ch0_raw < -max_allowed_bits) ch0_raw = -max_allowed_bits;\n            if (ch1_raw > max_allowed_bits)  ch1_raw = max_allowed_bits;\n            if (ch1_raw < -max_allowed_bits) ch1_raw = -max_allowed_bits;\n\n            // --- STEP 2: 3-SAMPLE MEDIAN FILTER ---\n            m0_2 = m0_1; m0_1 = m0_0; m0_0 = ch0_raw;\n            float s0_0 = m0_0; float s0_1 = m0_1; float s0_2 = m0_2;\n            if (s0_0 > s0_1) { temp0 = s0_0; s0_0 = s0_1; s0_1 = temp0; }\n            if (s0_1 > s0_2) { temp0 = s0_1; s0_1 = s0_2; s0_2 = temp0; }\n            if (s0_0 > s0_1) { temp0 = s0_0; s0_0 = s0_1; s0_1 = temp0; }\n            ch0_clean = s0_1;\n\n            m1_2 = m1_1; m1_1 = m1_0; m1_0 = ch1_raw;\n            float s1_0 = m1_0; float s1_1 = m1_1; float s1_2 = m1_2;\n            if (s1_0 > s1_1) { temp1 = s1_0; s1_0 = s1_1; s1_1 = temp1; }\n            if (s1_1 > s1_2) { temp1 = s1_1; s1_1 = s1_2; s1_2 = temp1; }\n            if (s1_0 > s1_1) { temp1 = s1_0; s1_0 = s1_1; s1_1 = temp1; }\n            ch1_clean = s1_1;\n\n            // --- STEP 3: EXPONENTIAL FILTER (STREAM LEVEL) ---\n            if (ch0_filt == 0.0) ch0_filt = ch0_clean;\n            if (ch1_filt == 0.0) ch1_filt = ch1_clean;\n\n            ch0_filt = ch0_filt + (ch0_clean - ch0_filt) * 0.125;\n            ch1_filt = ch1_filt + (ch1_clean - ch1_filt) * 0.125;\n\n            // --- STEP 4: MIN/MAX WINDOW CONTINUOUS ACCUMULATION ---\n            if (ch0_filt > max_ch0) max_ch0 = ch0_filt;\n            if (ch0_filt < min_ch0) min_ch0 = ch0_filt;\n            if (ch1_filt > max_ch1) max_ch1 = ch1_filt;\n            if (ch1_filt < min_ch1) min_ch1 = ch1_filt;\n\n            valid_samples++; // FIX: Successfully parsed and accumulated a clean point\n            start_idx = -1; \n        }\n    }\n}\n\n// --- STEP 5: WINDOW EVALUATION ENGINE ---\n// FIX: Condition updated to verify that valid samples exist for both channels\nif (((current_time_ms - start_time_ms) >= 50) && (valid_samples > 0) && (min_ch0 < 9000000.0) && (min_ch1 < 9000000.0)) {\n    window_ready = 1;\n\n    // Linear Bit-to-Voltage Transformations (LVDT - Channel 0)\n    out_LVDT_Min_V = (min_ch0 * VREF) / 8388607.0;\n    out_LVDT_Max_V = (max_ch0 * VREF) / 8388607.0;\n    raw_p2p_v = out_LVDT_Max_V - out_LVDT_Min_V;\n\n    // Linear Bit-to-Voltage Transformations (Piezo - Channel 1)\n    piezo_min_v = (min_ch1 * VREF) / 8388607.0;\n    piezo_max_v = (max_ch1 * VREF) / 8388607.0;\n    \n    // Assign Peak-to-Peak Voltage directly to output indicator (Matches Python logic)\n    out_Piezo_P2P = piezo_max_v - piezo_min_v;\n    \n    // Force scaling calculations using Voltage delta * Newtons/Volt Factor\n    raw_friction = out_Piezo_P2P * PIEZO_CAL_FACTOR + 0.44528;\n    raw_cof = raw_friction / NORMAL_FORCE;\n\n    // --- STEP 6: OUTPUT METRIC SMOOTHING (Low-Pass Filter Alpha = 0.05) ---\n    // Seed initial historical metrics if first loop iteration\n    if (hist_LVDT_P2P == 0.0) hist_LVDT_P2P = raw_p2p_v;\n    if (hist_Friction == 0.0) hist_Friction = raw_friction;\n    if (hist_COF == 0.0)      hist_COF = raw_cof;\n\n    // Apply exponential output dampening\n    hist_LVDT_P2P = hist_LVDT_P2P + (raw_p2p_v - hist_LVDT_P2P) * 0.05;\n    hist_Friction = hist_Friction + (raw_friction - hist_Friction) * 0.05; // Note: Can drop to 0.02 for more aggressive damping\n    hist_COF      = hist_COF + (raw_cof - hist_COF) * 0.05;\n\n    // Direct smoothed parameters out to UI Indicators\n    out_LVDT_P2P_V = hist_LVDT_P2P;\n    out_Friction_N = hist_Friction;\n    out_COF        = hist_COF;\n\n    // Reset tracking targets to extreme boundaries safely\n    min_ch0 = 9999999.0;\n    max_ch0 = -9999999.0;\n    min_ch1 = 9999999.0;\n    max_ch1 = -9999999.0;\n\n    valid_samples = 0; // FIX: Reset counter for next time frame\n    start_time_ms = current_time_ms;\n}"("raw_bytes"=w1948, "array_size"=w1947, "VREF"="VREF", "PIEZO_CAL_FACTOR"="PIEZO_CAL_FACTOR", "NORMAL_FORCE"="NORMAL_FORCE", "min_ch0"=w1943, "max_ch0"=w1942, "min_ch1"=w1941, "max_ch1"=w1940, "current_time_ms"=w1935, "start_time_ms"=w1934, "ch0_filt"=w1932, "ch1_filt"=w1931, "m0_0"=w1928, "m0_1"=w1927, "m0_2"=w1926, "m1_0"=w1925, "m1_1"=w1924, "m1_2"=w1923, "in_LVDT_Min_V"=w1916, "in_LVDT_Max_V"=w1909, "in_LVDT_P2P_V"=w1908, "in_Piezo_P2P"=w1907, "in_Friction_N"=w1906, "in_COF"=w1905, "hist_LVDT_P2P"=w1903, "hist_Friction"=w1902, "hist_COF"=w1901) -> ("window_ready"=→"Valid_data":dbl, "out_LVDT_Min_V"=w1915:dbl, "out_LVDT_Max_V"=w1914:dbl, "out_LVDT_P2P_V"=w1913:dbl, "out_Piezo_P2P"=w1912:dbl, "out_Friction_N"=w1911:dbl, "out_COF"=w1910:dbl, "min_ch0"=w1939:dbl, "max_ch0"=w1938:dbl, "min_ch1"=w1937:dbl, "max_ch1"=w1936:dbl, "start_time_ms"=w1933:u32, "ch0_filt"=w1930:dbl, "ch1_filt"=w1929:dbl, "m0_0"=w1922:dbl, "m0_1"=w1921:dbl, "m0_2"=w1920:dbl, "m1_0"=w1919:dbl, "m1_1"=w1918:dbl, "m1_2"=w1917:dbl, "hist_LVDT_P2P"=w1900:dbl, "hist_Friction"=w1899:dbl, "hist_COF"=w1898:dbl)
            "LVDT MIN" <- w1915
            "LVDT MAX" <- w1914
            "LVDT Peak" <- w1913
            "pizo raw" <- w1912
            "cof" <- w1910
            "Frictioin Force Raw" <- w1911
          }
        }
      }
      frame Error {
      }
    }
    n1634 = local read "Quit"() -> (w1829:bool)
  }
  n1635 = disable-structure shown="Disabled" {
    disable-tunnel: errorcluster {"status"=TRUE, "code"=0, "source"="Init"} ("error IO") -> [w1974 _]
    disable-tunnel: [w1972 _] -> w45
    frame Disabled {
      n1636 = while {
        shift-right: [w1990] -> w1976
        shift-left: _ -> [w1981]
        shift-right: [w1989] -> w1975
        shift-left: w1974 -> [w1983]
        tunnel: [w1978] -> w1972
        tunnel: [w1988] -> _
        i -> [w1988]
        stop <- w1978 stop-if-true
        n1637 = local read "Port 1a"() -> (w1984:bool)
        n1638 = local read "Port 3"() -> (w1985:bool)
        n1639 = local read "Com Port 1"() -> (w1982:refnum<visa-resource-name>)
        n1640 = Or(x=w1985, y=w1984) -> (x .or. y?=w1987:bool)
        n1641 = Unbundle(w1983) -> ("status"=→"Port 3":bool)  [unwired: 2 out]
        n1642 = Not Equal?(x=w1982, y=w1981) -> (x != y?=w1979:bool)
        n1643 = case shown="True" w1987 {
          frame False {
            w1993 = TRUE ("Visible")
            n1644 = property on="Port 1a" class="Bool (strict)"("Visible"=w1993) -> ()  [unwired: 2 in, 2 out]
            n1645 = property on="Port 3" class="Bool (strict)"("Visible"=w1993) -> ()  [unwired: 2 in, 2 out]
          }
          frame True {
            w1994 = TRUE ("Visible")
            n1646 = property on="Port 1a" class="Bool (strict)"("Visible"=w1994) -> ()  [unwired: 2 in, 2 out]
            n1647 = property on="Port 3" class="Bool (strict)"("Visible"=w1994) -> ()  [unwired: 2 in, 2 out]
          }
        }
        n1648 = Wait (ms)(milliseconds to wait=u32 40) -> ()  [unwired: 1 out]
        n1649 = case shown="True" w1979 {
          tunnel: [w1991 errorcluster {"status"=TRUE, "code"=0, "source"="Init"} ("error out")] -> w1980
          tunnel: w1983 -> [w1991 _]
          frame False {
          }
          frame True {
          }
        }
        n1650 = case shown="Error" w1980 {
          selector: w1980 -> [w2001 w2019]
          tunnel: [w2004 w2023] -> w1990
          tunnel: [w2003 w2017] -> w1989
          tunnel: w1981 -> [w2002 w2021]
          frame No Error {
            n1651 = property class="Instr"(reference=w2002, error in=w2001) -> (reference out=w1999:refnum<visa-resource-name>, error out=w2000:errorcluster, "Serial Settings:Number of Bytes at Serial Port"=w1996:u32)
            n1652 = Greater?(x=w1996, y=u32 5) -> (0:w1995:bool)
            n1653 = Not(x=w1995) -> (.not. x?=→"Port 1a":bool)
            n1654 = while {
              tunnel: [w2012] -> w2003
              tunnel: [w2011] -> w2004
              tunnel: w2000 -> [w2010]
              tunnel: w1999 -> [w2009]
              stop <- TRUE stop-if-true
              n1655 = property class="Instr" props=["Serial Settings:Number of Bytes at Serial Port"](reference=w2009, error in=w2010) -> (reference out=w2014:refnum<visa-resource-name>, error out=w2013:errorcluster)  [unwired: 1 out]
              n1656 = VISA Read(VISA resource name=w2014, byte count=u32 50, error in (no error)=w2013) -> (VISA resource name out=w2011:refnum<visa-resource-name>, read buffer=w2006:string, error out=w2012:errorcluster)  [unwired: 1 out]
              n1657 = Wait (ms)(milliseconds to wait=u32 5) -> ()  [unwired: 1 out]
            }
          }
          frame Error {
            w2029 = u16 0 items=["None", "XON/XOFF", "RTS/CTS", "XON/XOFF & RTS/CTS", "DTR/DSR", "XON/XOFF & DTR/DSR"] ("flow control (0:none)  2")
            w2027 = u16 10 items=["1.0"=10, "1.5"=15, "2.0"=20] ("stop bits 2")
            w2025 = u16 0 items=["None", "Odd", "Even", "Mark", "Space"] ("parity 2")
            w2026 = u32 10000  # timeout (10sec)
            n1658 = VISA Close(VISA resource name=w2021, error in (no error)=w2019) -> (error out=w2022:errorcluster)
            n1659 = local write "Port 1a"(FALSE ("Port 1a")) -> ()
            n1660 = local read "Com Port 1"() -> (w2016:refnum<visa-resource-name>)
            n1661 = call <vilib>:"Clear Errors.vi"("error in (no error)"=w2022) -> ("error out"=w2020:errorcluster)  [unwired: 5 in, 1 out]
            n1662 = call-poly "VISA Configure Serial Port"("VISA resource name"=w2016, "timeout (10sec)"=w2026, "baud rate (9600)"=u32 250000 ("baud rate  2"), "data bits (8)"=u16 8 ("data bits  2"), "parity (0:none)"=w2025, "error in (no error)"=w2020, "stop bits (10: 1 bit)"=w2027, "flow control (0:none)"=w2029) -> ("VISA resource name out"=w2030:refnum<visa-resource-name>, "error out"=w2031:errorcluster)  [unwired: 6 in]
            n1663 = flat-sequence {
              tunnel: w2030 -> [w2033]
              tunnel: w2031 -> [w2032]
              tunnel: [w2033] -> w2023
              tunnel: [w2032] -> w2017
              frame #0 {
                n1664 = Wait (ms)(milliseconds to wait=u32 50) -> ()  [unwired: 1 out]
              }
            }
            "Residual Uno" <- ""
          }
        }
        n1665 = local read "Quit"() -> (w1978:bool)
        "Error Uno" <- w1983
      }
      n1666 = VISA Close(VISA resource name=w1976, error in (no error)=w1975) -> (error out=w1973:errorcluster)
      n1667 = call <vilib>:"Clear Errors.vi"("error in (no error)"=w1973) -> ()  [unwired: 5 in, 2 out]
    }
    frame Enabled {
    }
  }
  n1668 = while {
    stop <- w2044 stop-if-true
    # "V0OLTAGE TO STROKE (peice vise calibration)"
    n1669 = local read "LVDT MIN"() -> (w2036:dbl)
    n1670 = local read "LVDT Peak"() -> (w2035:dbl)
    n1671 = Wait (ms)(milliseconds to wait=u32 10) -> ()  [unwired: 1 out]
    n1672 = formula code="// Dynamic Parameterized Linear Interpolation Node\n// Inputs: vpp_val, voltages (Array), distances (Array)\n// Outputs: stroke\n\nint i = 0;\nint segments = 11; // 12 points make 11 interpolation segments\n\n// 1. Lower Boundary Clamp\nif (vpp_val <= voltages[0]) {\n    stroke = distances[0];\n}\n// 2. Upper Boundary Clamp\nelse if (vpp_val >= voltages[segments]) {\n    stroke = distances[segments];\n}\n// 3. Dynamic Segment Search Loop\nelse {\n    stroke = distances[0]; // Fallback baseline\n    for (i = 0; i < segments; i++) {\n        if (vpp_val >= voltages[i] && vpp_val <= voltages[i+1]) {\n            // Standard linear interpolation formula using array lookups\n            stroke = distances[i] + (vpp_val - voltages[i]) * (distances[i+1] - distances[i]) / (voltages[i+1] - voltages[i]);\n            break; // Segment found, safely exit the loop\n        }\n    }\n}"("vpp_val"=w2035, "voltages"="calibration values", "distances"="STROKE") -> ("stroke"=→"LVDT STROKE":dbl)
    n1673 = local read "Calibration Tare Value"() -> (w2040:dbl)
    n1674 = local read "Calibration Tare"() -> (w2038:bool)
    n1675 = Subtract(x=w2036, y=w2040) -> (x-y=→"LVDT STROKE  Calibration":dbl)
    n1676 = case shown="True" w2038 {
      selector: w2038 -> [_ w2046]
      tunnel: w2036 -> [_ w2047]
      frame False {
      }
      frame True {
        n1677 = Not(x=w2046) -> (.not. x?=w2045:bool)
        n1678 = local write "Calibration Tare"(w2045) -> ()
        "Calibration Tare Value" <- w2047
      }
    }
    n1679 = local read "Quit"() -> (w2044:bool)
  }
  n1680 = while {
    stop <- w2070 stop-if-true
    n1681 = local read "Due read"() -> (w2068:string)
    n1682 = call <vilib>:"High Resolution Polling Wait.vi"("seconds to wait"=0.02) -> ()  [unwired: 10 in, 1 out]
    n1683 = local read "Frictioin Force Raw"() -> (w2050:dbl)
    n1684 = Spreadsheet String To Array(delimiter (Tab)=";", format string="", spreadsheet string=w2068, array type (2D Dbl)=string[] []) -> (array=w2065:string[])